vi "1D history with index.vi"   [LabVIEW 2021, in "Ring Buffer Strict Accessor Unit Tests.lvlib"]
uses:
  Ring Buffer Strict Accessor Unit Tests.lvlib
  Source/SubVIs/Endianess.ctl
  611bdaf6-9305-4b21-89ce-2c30f85c4112.vi
  feeae124-193a-4fa3-91dd-2bca20cfce72.vi
  423ce82f-b5fd-43ed-8c64-68510a1d3ff9.vi
  4892444c-7cdb-49e1-8809-bcb237467bd7.vi
  e30c749b-a05d-40c2-9d44-bf60a982eb2c.vi
  47326f7e-a0c6-4335-aeed-975c014db8ec.vi
  f586c412-da68-48e3-96db-4c5d284c8d62.vi
  1d5788e3-82fd-4730-bb71-cc7ffd3e5b8a.vi
  dea59858-e716-43e9-baf5-2617991b618f.vi
  611bdaf6-9305-4b21-89ce-2c30f85c4112.vi/4c2a6c61-f100-483c-8a49-51e57025a24c.vi
  611bdaf6-9305-4b21-89ce-2c30f85c4112.vi/e57bc314-87c7-4952-9bc8-929005dac297.vi
  <userlib>/bjustice/Ring Buffer for Time Series Data/API Poly.vi
  <userlib>/bjustice/Ring Buffer for Time Series Data/API/Write Array.vi
  feeae124-193a-4fa3-91dd-2bca20cfce72.vi/f2df9050-0eef-46c6-aff6-3ce3a8893ea5.vi
  423ce82f-b5fd-43ed-8c64-68510a1d3ff9.vi/17d75e1a-130a-47e0-8f2c-6c7d90b8ca77.vi
  <userlib>/bjustice/Ring Buffer for Time Series Data/API/Read Full Rotated Buffer.vi
  Source/SubVIs/Search for time to keep.vi
  Source/SubVIs/Index ByteArray.vi
  423ce82f-b5fd-43ed-8c64-68510a1d3ff9.vi/19bdd28a-0674-4be3-87bb-ec701e431d75.vi
  Source/SubVIs/error if empty buffer.vi
  4892444c-7cdb-49e1-8809-bcb237467bd7.vi/4c2a6c61-f100-483c-8a49-51e57025a24c.vi
  4892444c-7cdb-49e1-8809-bcb237467bd7.vi/e57bc314-87c7-4952-9bc8-929005dac297.vi
  e30c749b-a05d-40c2-9d44-bf60a982eb2c.vi/f2df9050-0eef-46c6-aff6-3ce3a8893ea5.vi
  47326f7e-a0c6-4335-aeed-975c014db8ec.vi/17d75e1a-130a-47e0-8f2c-6c7d90b8ca77.vi
  47326f7e-a0c6-4335-aeed-975c014db8ec.vi/19bdd28a-0674-4be3-87bb-ec701e431d75.vi
  f586c412-da68-48e3-96db-4c5d284c8d62.vi/4c2a6c61-f100-483c-8a49-51e57025a24c.vi
  f586c412-da68-48e3-96db-4c5d284c8d62.vi/e57bc314-87c7-4952-9bc8-929005dac297.vi
  1d5788e3-82fd-4730-bb71-cc7ffd3e5b8a.vi/f2df9050-0eef-46c6-aff6-3ce3a8893ea5.vi
  dea59858-e716-43e9-baf5-2617991b618f.vi/17d75e1a-130a-47e0-8f2c-6c7d90b8ca77.vi
  dea59858-e716-43e9-baf5-2617991b618f.vi/19bdd28a-0674-4be3-87bb-ec701e431d75.vi
  <userlib>/bjustice/Ring Buffer for Time Series Data/SubVIs/Split Values Array.vi
  <userlib>/bjustice/Ring Buffer for Time Series Data/SubVIs/Replace Values Array Multiple Timestamps.vi
  feeae124-193a-4fa3-91dd-2bca20cfce72.vi/f2df9050-0eef-46c6-aff6-3ce3a8893ea5.vi/63c583a5-c20f-4aba-9c90-661423dee4c4.vi
  feeae124-193a-4fa3-91dd-2bca20cfce72.vi/f2df9050-0eef-46c6-aff6-3ce3a8893ea5.vi/52385341-3d9c-45d2-aff5-e082a4793eb1.vi
  feeae124-193a-4fa3-91dd-2bca20cfce72.vi/f2df9050-0eef-46c6-aff6-3ce3a8893ea5.vi/37f29efa-f142-46b1-a185-f0098a95fbb6.vi
  feeae124-193a-4fa3-91dd-2bca20cfce72.vi/f2df9050-0eef-46c6-aff6-3ce3a8893ea5.vi/84b3d231-9afe-4b6e-afae-e0be43a31e4e.vi
  feeae124-193a-4fa3-91dd-2bca20cfce72.vi/f2df9050-0eef-46c6-aff6-3ce3a8893ea5.vi/c726271c-fc36-4bb7-8553-8945ec40c1cd.vi
  feeae124-193a-4fa3-91dd-2bca20cfce72.vi/f2df9050-0eef-46c6-aff6-3ce3a8893ea5.vi/a7b1d944-dc88-46f5-9d3e-305d46bbe1f6.vi
  feeae124-193a-4fa3-91dd-2bca20cfce72.vi/f2df9050-0eef-46c6-aff6-3ce3a8893ea5.vi/8abc4a6e-a1d2-4e85-879b-517e0ab55733.vi
  feeae124-193a-4fa3-91dd-2bca20cfce72.vi/f2df9050-0eef-46c6-aff6-3ce3a8893ea5.vi/bd347357-b475-4a03-9ac5-3b85ef11aecc.vi
  feeae124-193a-4fa3-91dd-2bca20cfce72.vi/f2df9050-0eef-46c6-aff6-3ce3a8893ea5.vi/391b36e9-a702-45e4-9499-3914f8833a58.vi
  feeae124-193a-4fa3-91dd-2bca20cfce72.vi/f2df9050-0eef-46c6-aff6-3ce3a8893ea5.vi/44155b33-c915-49ce-9e44-a66693aa70dd.vi
  feeae124-193a-4fa3-91dd-2bca20cfce72.vi/f2df9050-0eef-46c6-aff6-3ce3a8893ea5.vi/36977d53-dbe0-4dbc-b2ac-3dea4345b868.vi
  423ce82f-b5fd-43ed-8c64-68510a1d3ff9.vi/17d75e1a-130a-47e0-8f2c-6c7d90b8ca77.vi/bbb64351-fa28-4ac1-b583-44e271193ecd.vi
  <userlib>/bjustice/Ring Buffer for Time Series Data/SubVIs/Rotate Buffer.vi
  Source/SubVIs/Search for oldest time to keep.vi
  Source/SubVIs/Search for newest time to keep.vi
  Source/SubVIs/datatype byte size.vi
  Source/SubVIs/array sizes to number of points.vi
  423ce82f-b5fd-43ed-8c64-68510a1d3ff9.vi/19bdd28a-0674-4be3-87bb-ec701e431d75.vi/81c66277-30bd-484c-9c7c-9646f36721bb.vi
  423ce82f-b5fd-43ed-8c64-68510a1d3ff9.vi/19bdd28a-0674-4be3-87bb-ec701e431d75.vi/7ca10173-70f1-4bfb-9c4b-948090662032.vi
  423ce82f-b5fd-43ed-8c64-68510a1d3ff9.vi/19bdd28a-0674-4be3-87bb-ec701e431d75.vi/ea4aced9-3494-4b3f-b998-02af6afbdac4.vi
  423ce82f-b5fd-43ed-8c64-68510a1d3ff9.vi/19bdd28a-0674-4be3-87bb-ec701e431d75.vi/022c581c-5349-49df-98f9-5a038829ee63.vi
  423ce82f-b5fd-43ed-8c64-68510a1d3ff9.vi/19bdd28a-0674-4be3-87bb-ec701e431d75.vi/ed40bcc8-bbaa-4b61-9e1a-b4b75cf21b06.vi
  423ce82f-b5fd-43ed-8c64-68510a1d3ff9.vi/19bdd28a-0674-4be3-87bb-ec701e431d75.vi/f4b703c2-aaab-40a0-b3da-b0c22dc82d50.vi
  423ce82f-b5fd-43ed-8c64-68510a1d3ff9.vi/19bdd28a-0674-4be3-87bb-ec701e431d75.vi/1efa054f-b143-4d96-9f7e-584a7c6fa7fd.vi
  423ce82f-b5fd-43ed-8c64-68510a1d3ff9.vi/19bdd28a-0674-4be3-87bb-ec701e431d75.vi/b7c29f3f-256a-4401-af9d-aa15374df391.vi
  423ce82f-b5fd-43ed-8c64-68510a1d3ff9.vi/19bdd28a-0674-4be3-87bb-ec701e431d75.vi/2fb7b479-974d-4a18-8674-c4c8d9dc9a89.vi
  423ce82f-b5fd-43ed-8c64-68510a1d3ff9.vi/19bdd28a-0674-4be3-87bb-ec701e431d75.vi/faac7175-5814-4bb6-a961-a8db1f460653.vi
  423ce82f-b5fd-43ed-8c64-68510a1d3ff9.vi/19bdd28a-0674-4be3-87bb-ec701e431d75.vi/b6af2a6f-71a4-4cfe-837f-b196861458b0.vi
  e30c749b-a05d-40c2-9d44-bf60a982eb2c.vi/f2df9050-0eef-46c6-aff6-3ce3a8893ea5.vi/63c583a5-c20f-4aba-9c90-661423dee4c4.vi
  e30c749b-a05d-40c2-9d44-bf60a982eb2c.vi/f2df9050-0eef-46c6-aff6-3ce3a8893ea5.vi/52385341-3d9c-45d2-aff5-e082a4793eb1.vi
  e30c749b-a05d-40c2-9d44-bf60a982eb2c.vi/f2df9050-0eef-46c6-aff6-3ce3a8893ea5.vi/37f29efa-f142-46b1-a185-f0098a95fbb6.vi
  e30c749b-a05d-40c2-9d44-bf60a982eb2c.vi/f2df9050-0eef-46c6-aff6-3ce3a8893ea5.vi/84b3d231-9afe-4b6e-afae-e0be43a31e4e.vi
  e30c749b-a05d-40c2-9d44-bf60a982eb2c.vi/f2df9050-0eef-46c6-aff6-3ce3a8893ea5.vi/c726271c-fc36-4bb7-8553-8945ec40c1cd.vi
  e30c749b-a05d-40c2-9d44-bf60a982eb2c.vi/f2df9050-0eef-46c6-aff6-3ce3a8893ea5.vi/a7b1d944-dc88-46f5-9d3e-305d46bbe1f6.vi
  e30c749b-a05d-40c2-9d44-bf60a982eb2c.vi/f2df9050-0eef-46c6-aff6-3ce3a8893ea5.vi/8abc4a6e-a1d2-4e85-879b-517e0ab55733.vi
  e30c749b-a05d-40c2-9d44-bf60a982eb2c.vi/f2df9050-0eef-46c6-aff6-3ce3a8893ea5.vi/bd347357-b475-4a03-9ac5-3b85ef11aecc.vi
  e30c749b-a05d-40c2-9d44-bf60a982eb2c.vi/f2df9050-0eef-46c6-aff6-3ce3a8893ea5.vi/391b36e9-a702-45e4-9499-3914f8833a58.vi
  e30c749b-a05d-40c2-9d44-bf60a982eb2c.vi/f2df9050-0eef-46c6-aff6-3ce3a8893ea5.vi/44155b33-c915-49ce-9e44-a66693aa70dd.vi
  e30c749b-a05d-40c2-9d44-bf60a982eb2c.vi/f2df9050-0eef-46c6-aff6-3ce3a8893ea5.vi/36977d53-dbe0-4dbc-b2ac-3dea4345b868.vi
  47326f7e-a0c6-4335-aeed-975c014db8ec.vi/17d75e1a-130a-47e0-8f2c-6c7d90b8ca77.vi/bbb64351-fa28-4ac1-b583-44e271193ecd.vi
  47326f7e-a0c6-4335-aeed-975c014db8ec.vi/19bdd28a-0674-4be3-87bb-ec701e431d75.vi/81c66277-30bd-484c-9c7c-9646f36721bb.vi
  47326f7e-a0c6-4335-aeed-975c014db8ec.vi/19bdd28a-0674-4be3-87bb-ec701e431d75.vi/7ca10173-70f1-4bfb-9c4b-948090662032.vi
  47326f7e-a0c6-4335-aeed-975c014db8ec.vi/19bdd28a-0674-4be3-87bb-ec701e431d75.vi/ea4aced9-3494-4b3f-b998-02af6afbdac4.vi
  47326f7e-a0c6-4335-aeed-975c014db8ec.vi/19bdd28a-0674-4be3-87bb-ec701e431d75.vi/022c581c-5349-49df-98f9-5a038829ee63.vi
  47326f7e-a0c6-4335-aeed-975c014db8ec.vi/19bdd28a-0674-4be3-87bb-ec701e431d75.vi/ed40bcc8-bbaa-4b61-9e1a-b4b75cf21b06.vi
  47326f7e-a0c6-4335-aeed-975c014db8ec.vi/19bdd28a-0674-4be3-87bb-ec701e431d75.vi/f4b703c2-aaab-40a0-b3da-b0c22dc82d50.vi
  47326f7e-a0c6-4335-aeed-975c014db8ec.vi/19bdd28a-0674-4be3-87bb-ec701e431d75.vi/1efa054f-b143-4d96-9f7e-584a7c6fa7fd.vi
  47326f7e-a0c6-4335-aeed-975c014db8ec.vi/19bdd28a-0674-4be3-87bb-ec701e431d75.vi/b7c29f3f-256a-4401-af9d-aa15374df391.vi
  47326f7e-a0c6-4335-aeed-975c014db8ec.vi/19bdd28a-0674-4be3-87bb-ec701e431d75.vi/2fb7b479-974d-4a18-8674-c4c8d9dc9a89.vi
  47326f7e-a0c6-4335-aeed-975c014db8ec.vi/19bdd28a-0674-4be3-87bb-ec701e431d75.vi/faac7175-5814-4bb6-a961-a8db1f460653.vi
  47326f7e-a0c6-4335-aeed-975c014db8ec.vi/19bdd28a-0674-4be3-87bb-ec701e431d75.vi/b6af2a6f-71a4-4cfe-837f-b196861458b0.vi
  1d5788e3-82fd-4730-bb71-cc7ffd3e5b8a.vi/f2df9050-0eef-46c6-aff6-3ce3a8893ea5.vi/63c583a5-c20f-4aba-9c90-661423dee4c4.vi
  1d5788e3-82fd-4730-bb71-cc7ffd3e5b8a.vi/f2df9050-0eef-46c6-aff6-3ce3a8893ea5.vi/52385341-3d9c-45d2-aff5-e082a4793eb1.vi
  1d5788e3-82fd-4730-bb71-cc7ffd3e5b8a.vi/f2df9050-0eef-46c6-aff6-3ce3a8893ea5.vi/37f29efa-f142-46b1-a185-f0098a95fbb6.vi
  1d5788e3-82fd-4730-bb71-cc7ffd3e5b8a.vi/f2df9050-0eef-46c6-aff6-3ce3a8893ea5.vi/84b3d231-9afe-4b6e-afae-e0be43a31e4e.vi
  1d5788e3-82fd-4730-bb71-cc7ffd3e5b8a.vi/f2df9050-0eef-46c6-aff6-3ce3a8893ea5.vi/c726271c-fc36-4bb7-8553-8945ec40c1cd.vi
  1d5788e3-82fd-4730-bb71-cc7ffd3e5b8a.vi/f2df9050-0eef-46c6-aff6-3ce3a8893ea5.vi/a7b1d944-dc88-46f5-9d3e-305d46bbe1f6.vi
  1d5788e3-82fd-4730-bb71-cc7ffd3e5b8a.vi/f2df9050-0eef-46c6-aff6-3ce3a8893ea5.vi/8abc4a6e-a1d2-4e85-879b-517e0ab55733.vi
  1d5788e3-82fd-4730-bb71-cc7ffd3e5b8a.vi/f2df9050-0eef-46c6-aff6-3ce3a8893ea5.vi/bd347357-b475-4a03-9ac5-3b85ef11aecc.vi
  1d5788e3-82fd-4730-bb71-cc7ffd3e5b8a.vi/f2df9050-0eef-46c6-aff6-3ce3a8893ea5.vi/391b36e9-a702-45e4-9499-3914f8833a58.vi
  1d5788e3-82fd-4730-bb71-cc7ffd3e5b8a.vi/f2df9050-0eef-46c6-aff6-3ce3a8893ea5.vi/44155b33-c915-49ce-9e44-a66693aa70dd.vi
  1d5788e3-82fd-4730-bb71-cc7ffd3e5b8a.vi/f2df9050-0eef-46c6-aff6-3ce3a8893ea5.vi/36977d53-dbe0-4dbc-b2ac-3dea4345b868.vi
  dea59858-e716-43e9-baf5-2617991b618f.vi/17d75e1a-130a-47e0-8f2c-6c7d90b8ca77.vi/bbb64351-fa28-4ac1-b583-44e271193ecd.vi
  dea59858-e716-43e9-baf5-2617991b618f.vi/19bdd28a-0674-4be3-87bb-ec701e431d75.vi/81c66277-30bd-484c-9c7c-9646f36721bb.vi
  dea59858-e716-43e9-baf5-2617991b618f.vi/19bdd28a-0674-4be3-87bb-ec701e431d75.vi/7ca10173-70f1-4bfb-9c4b-948090662032.vi
  dea59858-e716-43e9-baf5-2617991b618f.vi/19bdd28a-0674-4be3-87bb-ec701e431d75.vi/ea4aced9-3494-4b3f-b998-02af6afbdac4.vi
  dea59858-e716-43e9-baf5-2617991b618f.vi/19bdd28a-0674-4be3-87bb-ec701e431d75.vi/022c581c-5349-49df-98f9-5a038829ee63.vi
  dea59858-e716-43e9-baf5-2617991b618f.vi/19bdd28a-0674-4be3-87bb-ec701e431d75.vi/ed40bcc8-bbaa-4b61-9e1a-b4b75cf21b06.vi
  dea59858-e716-43e9-baf5-2617991b618f.vi/19bdd28a-0674-4be3-87bb-ec701e431d75.vi/f4b703c2-aaab-40a0-b3da-b0c22dc82d50.vi
  dea59858-e716-43e9-baf5-2617991b618f.vi/19bdd28a-0674-4be3-87bb-ec701e431d75.vi/1efa054f-b143-4d96-9f7e-584a7c6fa7fd.vi
  dea59858-e716-43e9-baf5-2617991b618f.vi/19bdd28a-0674-4be3-87bb-ec701e431d75.vi/b7c29f3f-256a-4401-af9d-aa15374df391.vi
  dea59858-e716-43e9-baf5-2617991b618f.vi/19bdd28a-0674-4be3-87bb-ec701e431d75.vi/2fb7b479-974d-4a18-8674-c4c8d9dc9a89.vi
  dea59858-e716-43e9-baf5-2617991b618f.vi/19bdd28a-0674-4be3-87bb-ec701e431d75.vi/faac7175-5814-4bb6-a961-a8db1f460653.vi
  dea59858-e716-43e9-baf5-2617991b618f.vi/19bdd28a-0674-4be3-87bb-ec701e431d75.vi/b6af2a6f-71a4-4cfe-837f-b196861458b0.vi
  <userlib>/bjustice/Ring Buffer for Time Series Data/SubVIs/Enforce array size multiple timestamps.vi
  Source/API/New.vi
  <vilib>/Utility/error.llb/Error Cluster From Error Code.vi
  <vilib>/Utility/error.llb/Trim Whitespace.vi
  <vilib>/addons/_JKI Toolkits/Caraya/classes/Assert/Assert Not Error.vi
  <vilib>/addons/_JKI Toolkits/Caraya/classes/Assert/Assert True.vi
  <vilib>/addons/_JKI Toolkits/Caraya/classes/Assert/Assert Equal Value_Variant.vi
  Source/Ring Buffer Strict Accessor.lvlib
  <vilib>/addons/_JKI Toolkits/Caraya/classes/Assert/Assert.lvclass
  <vilib>/addons/_JKI Toolkits/Caraya/classes/Test/Test.lvclass
types:
  T1 = typedef "Ring Buffer Strict Accessor.lvlib/Endianess.ctl" = enum16{"big-endian", "little-endian"}
  T2 = typedef "Ring Buffer Strict Accessor.lvlib/RingBufferHandle.ctl" = cluster{"Ring buffer DVR":refnum<data-value>, "Data Type":T3, "Size(s)":i32[], "Endianess":T1, "Buffer Size (#timestamps) [init]":i32}
  T3 = typedef "Ring Buffer Strict Accessor.lvlib/DataType.ctl" = enum16{"uint8", "uint16", "uint32", "uint64", "int8", "int16", "int32", "int64", "float", "double", "extended"}
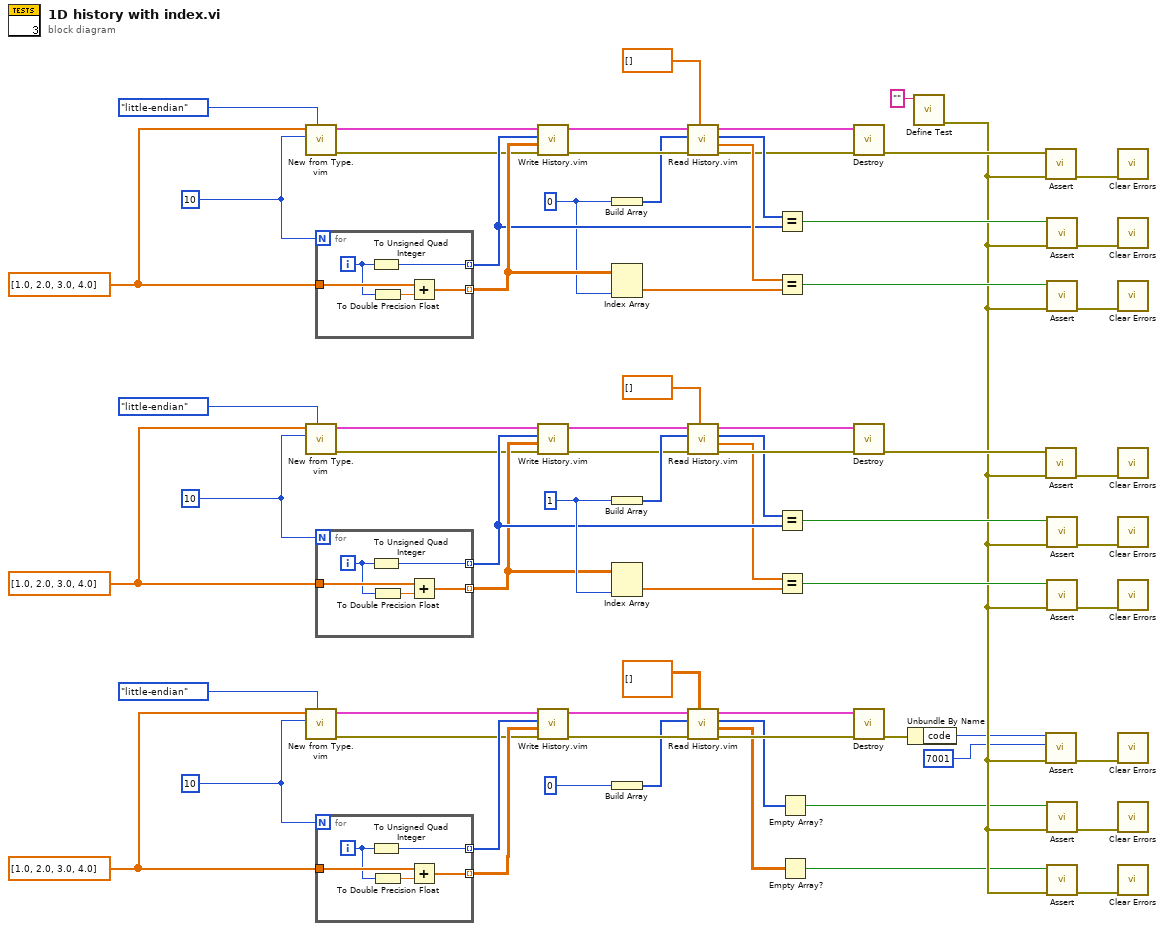
[diagram p0: block diagram]
diagram:
  w1 = 10 ("Buffer Size (#timestamps)")
  w3 = dbl[] [1.0, 2.0, 3.0, 4.0]
  w53 = 1 ("index")
  w6 = 10 ("Buffer Size (#timestamps)")
  w8 = dbl[] [1.0, 2.0, 3.0, 4.0]
  w54 = 0 ("index")
  w11 = 10 ("Buffer Size (#timestamps)")
  w12 = dbl[] [1.0, 2.0, 3.0, 4.0]
  n1 = call "New from Type.vim"("Endianess"=Endianess."little-endian", "Buffer Size (#timestamps)"=w11, "LV type (array size cannot be empty)"=w12) -> ("error out"=w13:errorcluster, "Ring Buffer"=w14:T2)  [unwired: 7 in]
  n2 = call "New from Type.vim"("Endianess"=Endianess."little-endian", "Buffer Size (#timestamps)"=w6, "LV type (array size cannot be empty)"=w8) -> ("error out"=w9:errorcluster, "Ring Buffer"=w10:T2)  [unwired: 7 in]
  n3 = call "New from Type.vim"("Endianess"=Endianess."little-endian", "Buffer Size (#timestamps)"=w1, "LV type (array size cannot be empty)"=w3) -> ("error out"=w4:errorcluster, "Ring Buffer"=w5:T2)  [unwired: 7 in]
  n4 = for {
    N: w11 -> [_]
    tunnel: w12 -> [w77]
    tunnel: [w76] -> w60 mode=indexing
    tunnel: [w75] -> w55 mode=indexing
    i -> [w74]
    n5 = To Unsigned Quad Integer(1:w74) -> (0:w75:u64)
    n6 = To Double Precision Float(number=w74) -> (double precision float=w73:dbl)
    n7 = Add(x=w77, y=w73) -> (x+y=w76:dbl[])
  }
  n8 = for {
    N: w6 -> [_]
    tunnel: w8 -> [w82]
    tunnel: [w81] -> w47 mode=indexing
    tunnel: [w80] -> w52 mode=indexing
    i -> [w79]
    n9 = To Unsigned Quad Integer(1:w79) -> (0:w80:u64)
    n10 = To Double Precision Float(number=w79) -> (double precision float=w78:dbl)
    n11 = Add(x=w82, y=w78) -> (x+y=w81:dbl[])
  }
  n12 = for {
    N: w1 -> [_]
    tunnel: w3 -> [w87]
    tunnel: [w86] -> w29 mode=indexing
    tunnel: [w85] -> w25 mode=indexing
    i -> [w84]
    n13 = To Unsigned Quad Integer(1:w84) -> (0:w85:u64)
    n14 = To Double Precision Float(number=w84) -> (double precision float=w83:dbl)
    n15 = Add(x=w87, y=w83) -> (x+y=w86:dbl[])
  }
  n16 = call "Write History.vim"("error in (no error)"=w13, "LV DataType"=w60, "Timestamps"=w55, "Ring Buffer"=w14) -> ("error out"=w67:errorcluster, "Ring Buffer"=w72:T2)  [unwired: 6 in]
  n17 = call "Write History.vim"("error in (no error)"=w9, "LV DataType"=w47, "Timestamps"=w52, "Ring Buffer"=w10) -> ("error out"=w41:errorcluster, "Ring Buffer"=w36:T2)  [unwired: 6 in]
  n18 = call "Write History.vim"("error in (no error)"=w4, "LV DataType"=w29, "Timestamps"=w25, "Ring Buffer"=w5) -> ("error out"=w32:errorcluster, "Ring Buffer"=w35:T2)  [unwired: 6 in]
  n19 = Build Array(w54) -> (w61:i32[])
  n20 = Index Array(array=w60, index (col)=w54) -> (element=w59:dbl[])  [unwired: 1 in]
  n21 = Build Array(w53) -> (w46:i32[])
  n22 = Index Array(array=w47, index (col)=w53) -> (element=w48:dbl[])  [unwired: 1 in]
  n23 = Build Array(0 ("index")) -> (w30:i32[])
  n24 = call "Read History.vim"("data type"=dbl[] [], "error in (no error)"=w67, "index"=w61, "Ring Buffer"=w72) -> ("error out"=w66:errorcluster, "Values"=w68:dbl[], "Timestamps"=w69:u64[], "Ring Buffer"=w71:T2)  [unwired: 4 in]
  n25 = call "Read History.vim"("data type"=dbl[] [], "error in (no error)"=w41, "index"=w46, "Ring Buffer"=w36) -> ("error out"=w42:errorcluster, "Values"=w40:dbl[], "Timestamps"=w39:u64[], "Ring Buffer"=w37:T2)  [unwired: 4 in]
  n26 = call "Read History.vim"("data type"=dbl[][] [], "error in (no error)"=w32, "index"=w30, "Ring Buffer"=w35) -> ("error out"=w31:errorcluster, "Values"=w20:dbl[][], "Timestamps"=w22:u64[], "Ring Buffer"=w34:T2)  [unwired: 4 in]
  n27 = Equal?(x=w69, y=w55) -> (x = y?=w65:bool)
  n28 = Equal?(x=w68, y=w59) -> (x = y?=w64:bool)
  n29 = Equal?(x=w39, y=w52) -> (x = y?=w43:bool)
  n30 = Equal?(x=w40, y=w48) -> (x = y?=w44:bool)
  n31 = Empty Array?(array=w22) -> (empty?=w21:bool)
  n32 = Empty Array?(array=w20) -> (empty?=w19:bool)
  n33 = call "Destroy.vi"("error in (no error)"=w66, "Ring Buffer"=w71) -> ("error out"=w63:errorcluster)  [unwired: 9 in]
  n34 = call "Destroy.vi"("error in (no error)"=w42, "Ring Buffer"=w37) -> ("error out"=w45:errorcluster)  [unwired: 9 in]
  n35 = call "Destroy.vi"("error in (no error)"=w31, "Ring Buffer"=w34) -> ("error out"=w18:errorcluster)  [unwired: 9 in]
  n36 = Unbundle By Name(w18) -> ("code"=w17:i32)
  n37 = call <vilib>:"Define Test.vi"("Label (VI Title)"="") -> ("error out"=w23:errorcluster)  [unwired: 9 in, 1 out]
  n38 = call-poly <vilib>:"Assert.vi"("error in (no error)"=w23, "Not Error?"=w63) -> ("error out"=w58:errorcluster)  [unwired: 8 in, 1 out]
  n39 = call-poly <vilib>:"Assert.vi"("error in (no error)"=w23, "Not Error?"=w45) -> ("error out"=w49:errorcluster)  [unwired: 8 in, 1 out]
  n40 = call-poly <vilib>:"Assert.vi"("error in (no error)"=w23, "Y"=7001 ("code"), "X"=w17) -> ("error out"=w28:errorcluster)  [unwired: 7 in, 1 out]
  n41 = call-poly <vilib>:"Assert.vi"("error in (no error)"=w23, "True?"=w65) -> ("error out"=w57:errorcluster)  [unwired: 8 in, 1 out]
  n42 = call-poly <vilib>:"Assert.vi"("error in (no error)"=w23, "True?"=w64) -> ("error out"=w56:errorcluster)  [unwired: 8 in, 1 out]
  n43 = call-poly <vilib>:"Assert.vi"("error in (no error)"=w23, "True?"=w43) -> ("error out"=w50:errorcluster)  [unwired: 8 in, 1 out]
  n44 = call-poly <vilib>:"Assert.vi"("error in (no error)"=w23, "True?"=w44) -> ("error out"=w51:errorcluster)  [unwired: 8 in, 1 out]
  n45 = call-poly <vilib>:"Assert.vi"("error in (no error)"=w23, "True?"=w21) -> ("error out"=w27:errorcluster)  [unwired: 8 in, 1 out]
  n46 = call-poly <vilib>:"Assert.vi"("error in (no error)"=w23, "True?"=w19) -> ("error out"=w26:errorcluster)  [unwired: 8 in, 1 out]
  n47 = call <vilib>:"Clear Errors.vi"("error in (no error)"=w58) -> ()  [unwired: 5 in, 2 out]
  n48 = call <vilib>:"Clear Errors.vi"("error in (no error)"=w57) -> ()  [unwired: 5 in, 2 out]
  n49 = call <vilib>:"Clear Errors.vi"("error in (no error)"=w56) -> ()  [unwired: 5 in, 2 out]
  n50 = call <vilib>:"Clear Errors.vi"("error in (no error)"=w49) -> ()  [unwired: 5 in, 2 out]
  n51 = call <vilib>:"Clear Errors.vi"("error in (no error)"=w50) -> ()  [unwired: 5 in, 2 out]
  n52 = call <vilib>:"Clear Errors.vi"("error in (no error)"=w51) -> ()  [unwired: 5 in, 2 out]
  n53 = call <vilib>:"Clear Errors.vi"("error in (no error)"=w28) -> ()  [unwired: 5 in, 2 out]
  n54 = call <vilib>:"Clear Errors.vi"("error in (no error)"=w27) -> ()  [unwired: 5 in, 2 out]
  n55 = call <vilib>:"Clear Errors.vi"("error in (no error)"=w26) -> ()  [unwired: 5 in, 2 out]
